vi "Dresden R2R Sputter 03.02.2018 IY24.vi"() -> ()   [LabVIEW 2009] (continued)
              frame #0 {
                n9135 = Wait (ms)(milliseconds to wait=i32? 100) -> ()  [unwired: 1 out]
              }
            }
            "Tp4_stop_cmnd" <- T/1 ("Tp4_stop_cmnd")
          }
          frame #3 {
            # "Address"
            n9136 = Multiply(x="Low_speed_value 4", y=data[16B]) -> (x*y=w14842)
            n9137 = To Unsigned Long Integer(number=w14842) -> (unsigned 32bit integer=w14841)
            n9138 = Number To Decimal String(number=w14841) -> (decimal integer string=w14839)  [unwired: 1 out]
            n9139 = String Length(string=w14839) -> (length=w14840)
            n9140 = case shown="0, Default" w14840 {
              tunnel: w14839 -> [_ w14868 w14871 w14872]
              tunnel: [data[5B] w14867 w14870 w14872] -> w14838
              frame #0 {
              }
              frame #1 {
                n9141 = Concatenate Strings(w14868, "00" ("string")) -> (w14867)
              }
              frame #2 {
                n9142 = Concatenate Strings(w14871, "0" ("string")) -> (w14870)
              }
              frame #3 {
              }
            }
            n9143 = Concatenate Strings("004" ("write buffer"), "10" ("string"), "707" ("string"), "06" ("string"), "00" ("string"), w14838) -> (w14852)
            n9144 = String To Byte Array(string=w14852) -> (unsigned byte array=w14857)
            n9145 = for {
              tunnel: w14857 -> [w14886] mode=indexing
              shift-right: [w14884] -> w14859
              shift-left: i16? 0 -> [w14885]
              n9146 = Add(x=w14886, y=w14885) -> (x+y=w14884)
            }
            n9147 = Number To Decimal String(number=w14859) -> (decimal integer string=w14854)  [unwired: 1 in]
            n9148 = String Length(string=w14854) -> (length=w14855)
            n9149 = case shown="0, Default" w14855 {
              tunnel: w14854 -> [_ w14879 w14882 w14883]
              tunnel: [data[5B] w14877 w14880 w14883] -> w14853
              frame #0 {
              }
              frame #1 {
                n9150 = Concatenate Strings("00" ("string"), w14879) -> (w14877)
              }
              frame #2 {
                n9151 = Concatenate Strings("0" ("string"), w14882) -> (w14880)
              }
              frame #3 {
              }
            }
            n9152 = Concatenate Strings(w14852, w14853, "\n") -> (w14849)
            n9153 = VISA Write(VISA resource name=w14848, write buffer=w14849, error in (no error)=w14847) -> (VISA resource name out=w14851, error out=w14850)  [unwired: 1 out]
            n9154 = stacked-sequence {
              tunnel: [w14875] -> w14846
              tunnel: w14851 -> [w14875]
              tunnel: [w14874] -> w14845
              tunnel: w14850 -> [w14874]
              frame #0 {
                n9155 = Wait (ms)(milliseconds to wait=i32? 100) -> ()  [unwired: 1 out]
              }
            }
          }
          frame #4 {
            # "Cheksum 3 haneli olmalı"
            # "Address"
            n9156 = Concatenate Strings("004" ("write buffer"), "10" ("string"), "026" ("string"), "03" ("string"), "001" ("string")) -> (w14894)
            n9157 = String To Byte Array(string=w14894) -> (unsigned byte array=w14899)
            n9158 = for {
              tunnel: w14899 -> [w14920] mode=indexing
              shift-right: [w14918] -> w14901
              shift-left: i16? 0 -> [w14919]
              n9159 = Add(x=w14920, y=w14919) -> (x+y=w14918)
            }
            n9160 = Number To Decimal String(number=w14901) -> (decimal integer string=w14896)  [unwired: 1 in]
            n9161 = String Length(string=w14896) -> (length=w14897)
            n9162 = case shown="0, Default" w14897 {
              tunnel: w14896 -> [_ w14913 w14916 w14917]
              tunnel: [data[5B] w14911 w14914 w14917] -> w14895
              frame #0 {
              }
              frame #1 {
                n9163 = Concatenate Strings("00" ("string"), w14913) -> (w14911)
              }
              frame #2 {
                n9164 = Concatenate Strings("0" ("string"), w14916) -> (w14914)
              }
              frame #3 {
              }
            }
            n9165 = Concatenate Strings(w14894, w14895, "\n") -> (w14891)
            n9166 = VISA Write(VISA resource name=w14890, write buffer=w14891, error in (no error)=w14889) -> (VISA resource name out=w14893, error out=w14892)  [unwired: 1 out]
            n9167 = stacked-sequence {
              tunnel: [w14909] -> w14888
              tunnel: w14893 -> [w14909]
              tunnel: [w14908] -> w14887
              tunnel: w14892 -> [w14908]
              frame #0 {
                n9168 = Wait (ms)(milliseconds to wait=i32? 100) -> ()  [unwired: 1 out]
              }
            }
          }
          frame #5 {
            # "Cheksum 3 haneli olmalı"
            # "Address"
            n9169 = Concatenate Strings("004" ("write buffer"), "10" ("string"), "026" ("string"), "03" ("string"), "000" ("string")) -> (w14928)
            n9170 = String To Byte Array(string=w14928) -> (unsigned byte array=w14933)
            n9171 = for {
              tunnel: w14933 -> [w14954] mode=indexing
              shift-right: [w14952] -> w14935
              shift-left: i16? 0 -> [w14953]
              n9172 = Add(x=w14954, y=w14953) -> (x+y=w14952)
            }
            n9173 = Number To Decimal String(number=w14935) -> (decimal integer string=w14930)  [unwired: 1 in]
            n9174 = String Length(string=w14930) -> (length=w14931)
            n9175 = case shown="0, Default" w14931 {
              tunnel: w14930 -> [_ w14947 w14950 w14951]
              tunnel: [data[5B] w14945 w14948 w14951] -> w14929
              frame #0 {
              }
              frame #1 {
                n9176 = Concatenate Strings("00" ("string"), w14947) -> (w14945)
              }
              frame #2 {
                n9177 = Concatenate Strings("0" ("string"), w14950) -> (w14948)
              }
              frame #3 {
              }
            }
            n9178 = Concatenate Strings(w14928, w14929, "\n") -> (w14925)
            n9179 = VISA Write(VISA resource name=w14924, write buffer=w14925, error in (no error)=w14923) -> (VISA resource name out=w14927, error out=w14926)  [unwired: 1 out]
            n9180 = stacked-sequence {
              tunnel: [w14943] -> w14922
              tunnel: w14927 -> [w14943]
              tunnel: [w14942] -> w14921
              tunnel: w14926 -> [w14942]
              frame #0 {
                n9181 = Wait (ms)(milliseconds to wait=i32? 100) -> ()  [unwired: 1 out]
              }
            }
          }
          frame #6 {
            # "Cheksum 3 haneli olmalı"
            # "Address"
            n9182 = Concatenate Strings("004" ("write buffer"), "10" ("string"), "023" ("string"), "06" ("string"), "111111" ("string")) -> (w14962)
            n9183 = String To Byte Array(string=w14962) -> (unsigned byte array=w14967)
            n9184 = for {
              tunnel: w14967 -> [w14988] mode=indexing
              shift-right: [w14986] -> w14969
              shift-left: i16? 0 -> [w14987]
              n9185 = Add(x=w14988, y=w14987) -> (x+y=w14986)
            }
            n9186 = Number To Decimal String(number=w14969) -> (decimal integer string=w14964)  [unwired: 1 in]
            n9187 = String Length(string=w14964) -> (length=w14965)
            n9188 = case shown="0, Default" w14965 {
              tunnel: w14964 -> [_ w14981 w14984 w14985]
              tunnel: [data[5B] w14979 w14982 w14985] -> w14963
              frame #0 {
              }
              frame #1 {
                n9189 = Concatenate Strings("00" ("string"), w14981) -> (w14979)
              }
              frame #2 {
                n9190 = Concatenate Strings("0" ("string"), w14984) -> (w14982)
              }
              frame #3 {
              }
            }
            n9191 = Concatenate Strings(w14962, w14963, "\n") -> (w14959)
            n9192 = VISA Write(VISA resource name=w14958, write buffer=w14959, error in (no error)=w14957) -> (VISA resource name out=w14961, error out=w14960)  [unwired: 1 out]
            n9193 = stacked-sequence {
              tunnel: [w14977] -> w14956
              tunnel: w14961 -> [w14977]
              tunnel: [w14976] -> w14955
              tunnel: w14960 -> [w14976]
              frame #0 {
                n9194 = Wait (ms)(milliseconds to wait=i32? 100) -> ()  [unwired: 1 out]
              }
            }
          }
          frame #7 {
            # "Cheksum 3 haneli olmalı"
            # "Address"
            n9195 = Concatenate Strings("004" ("write buffer"), "10" ("string"), "023" ("string"), "06" ("string"), "000000" ("string")) -> (w14996)
            n9196 = String To Byte Array(string=w14996) -> (unsigned byte array=w15001)
            n9197 = for {
              tunnel: w15001 -> [w15022] mode=indexing
              shift-right: [w15020] -> w15003
              shift-left: i16? 0 -> [w15021]
              n9198 = Add(x=w15022, y=w15021) -> (x+y=w15020)
            }
            n9199 = Number To Decimal String(number=w15003) -> (decimal integer string=w14998)  [unwired: 1 in]
            n9200 = String Length(string=w14998) -> (length=w14999)
            n9201 = case shown="0, Default" w14999 {
              tunnel: w14998 -> [_ w15015 w15018 w15019]
              tunnel: [data[5B] w15013 w15016 w15019] -> w14997
              frame #0 {
              }
              frame #1 {
                n9202 = Concatenate Strings("00" ("string"), w15015) -> (w15013)
              }
              frame #2 {
                n9203 = Concatenate Strings("0" ("string"), w15018) -> (w15016)
              }
              frame #3 {
              }
            }
            n9204 = Concatenate Strings(w14996, w14997, "\n") -> (w14993)
            n9205 = VISA Write(VISA resource name=w14992, write buffer=w14993, error in (no error)=w14991) -> (VISA resource name out=w14995, error out=w14994)  [unwired: 1 out]
            n9206 = stacked-sequence {
              tunnel: [w15011] -> w14990
              tunnel: w14995 -> [w15011]
              tunnel: [w15010] -> w14989
              tunnel: w14994 -> [w15010]
              frame #0 {
                n9207 = Wait (ms)(milliseconds to wait=i32? 100) -> ()  [unwired: 1 out]
              }
            }
          }
        }
      }
    }
  }
  n9208 = while {
    tunnel: w749 -> [w15026]
    tunnel: w775 -> [w15025]
    tunnel: [w15029] -> w774
    tunnel: [w15024] -> w743
    tunnel: "milliseconds to wait 2" -> [w15023]
    stop <- FALSE stop-if-true
    n9209 = stacked-sequence {
      tunnel: w15025 -> [w15034 _]
      tunnel: [w15033 _] -> w15029
      tunnel: w15026 -> [w15032 _]
      tunnel: [w15031 _] -> w15024
      tunnel: w15023 -> [w15030 _]
      frame #0 {
        n9210 = stacked-sequence {
          tunnel: w15032 -> [w15045 _ _ _ _ _ _ _ _]
          tunnel: w15034 -> [w15044 _ _ _ _ _ _ _ _]
          tunnel: [_ _ _ w15171 _ _ _ _ _] -> w15031
          tunnel: [_ _ _ w15169 _ _ _ _ _] -> w15033
          tunnel: w15030 -> [_ _ w15168 _ w15249 _ w15409 _ w15446]
          frame #0 {
            # "Digital I/O & Analog \nOutput Part"
            n9211 = disable-structure shown="Enabled" {
              disable-tunnel: w15045 -> [w15146 w15148]
              disable-tunnel: w15044 -> [w15145 w15147]
              disable-tunnel: [w15127 w15148] -> w15043
              disable-tunnel: [w15126 w15147] -> w15042
              frame #0 {
                n9212 = call-poly <vilib>:"MB Serial Master Query (poly).vi"("VISA resource name"=w15146, "Starting Address"=u16 0, "Quantity"=u16 8, "error in"=w15145, "Serial Parameters"=T39 {"Mode"=enum."RTU", "Slave Address"=1}) -> ("VISA resource name out"=w15127:refnum<visa-resource-name>, "Discrete Inputs"=w15135:bool[], "error out"=w15126:errorcluster)  [unwired: 1 in, 11 out]
                n9213 = Index Array(array=w15135, index=5) -> (element=w15125:bool)
                "Ch1_Pl_vbv_di" <- w15125
                n9214 = Index Array(array=w15135, index=6) -> (element=w15130:bool)
                "Ch1_Pl_atm_di" <- w15130
                n9215 = Index Array(array=w15135, index=7) -> (element=w15123:bool)
                "Ch1_Cc_on_off_di" <- w15123
                n9216 = Index Array(array=w15135, index=0) -> (element=w15133:bool)
                "Ch1_Mp_di" <- w15133
                n9217 = Index Array(array=w15135, index=1) -> (element=w15129:bool)
                "Ch1_Tp_bv_di" <- w15129
                n9218 = Index Array(array=w15135, index=2) -> (element=w15124:bool)
                "Ch1_Bg_bv_di" <- w15124
                n9219 = Index Array(array=w15135, index=3) -> (element=w15132:bool)
                "Ch1_Ch_vbv_di" <- w15132
                n9220 = Index Array(array=w15135, index=4) -> (element=w15131:bool)
                "Ch1_Ch_atm_di" <- w15131
                n9221 = local write "ch1_bg_bv_on_top"(w15124) -> ()
                n9222 = local write "Ch1_Ch_vbv_on"(w15132) -> ()
                n9223 = local write "ch4_atm_on_top"(w15131) -> ()
                n9224 = local write "Ch1_Ch_atm_on"(w15131) -> ()
                n9225 = local write "Ch1_Mp_on"(w15133) -> ()
                n9226 = local write "Ch1_Tp_bv_on"(w15129) -> ()
                n9227 = local write "Ch1_Bg_bv_on"(w15124) -> ()
                n9228 = local write "Ch1_Pl_vbv_on"(w15125) -> ()
                n9229 = local write "Ch1_Pl_atm_on"(w15130) -> ()
                n9230 = local write "Ch1_Ch_cc_on"(w15123) -> ()
                n9231 = local write "ch1_cc_on_top"(w15123) -> ()
              }
              frame #1 {
              }
            }
            n9232 = disable-structure shown="Enabled" {
              disable-tunnel: w15043 -> [w15104 w15122]
              disable-tunnel: w15042 -> [w15102 w15121]
              disable-tunnel: [w15101 w15122] -> w15041
              disable-tunnel: [w15100 w15121] -> w15040
              frame #0 {
                n9233 = call-poly <vilib>:"MB Serial Master Query (poly).vi"("VISA resource name"=w15104, "Starting Address"=u16 0, "Quantity"=u16 8, "error in"=w15102, "Serial Parameters"=T39 {"Mode"=enum."RTU", "Slave Address"=2}) -> ("VISA resource name out"=w15101:refnum<visa-resource-name>, "Discrete Inputs"=w15114:bool[], "error out"=w15100:errorcluster)  [unwired: 1 in, 11 out]
                n9234 = Index Array(array=w15114, index=5) -> (element=w15098:bool)
                "Ch1_Cst_fix_down_di" <- w15098
                n9235 = Index Array(array=w15114, index=6) -> (element=→"Ch1_Pet_cool_up_di":bool)
                n9236 = Index Array(array=w15114, index=7) -> (element=→"Ch1_Pet_cool_down_di":bool)
                n9237 = Index Array(array=w15114, index=0) -> (element=w15099:bool)
                "Ch1_Sov_Ar_di" <- w15099
                n9238 = Index Array(array=w15114, index=1) -> (element=w15097:bool)
                "Ch1_Trns_gv_open_di" <- w15097
                n9239 = Index Array(array=w15114, index=2) -> (element=→"Ch1_Trns_gv_close_di":bool)
                n9240 = Index Array(array=w15114, index=3) -> (element=→"Ch1_2_3_di":bool)
                n9241 = Index Array(array=w15114, index=4) -> (element=→"Ch1_Cst_fix_up_di":bool)
                n9242 = local write "chamber 1 top piston open ch1"(w15098) -> ()
                n9243 = local write "ch1_sov_Ar_on_top"(w15099) -> ()
                n9244 = local write "gv front open ch1_2"(w15097) -> ()
                n9245 = local write "Trns_gv_1_2_on"(w15097) -> ()
                n9246 = local write "gv top open ch1"(w15097) -> ()
                n9247 = local write "gv front open_ch2_1"(w15097) -> ()
                n9248 = local write "gv top_open_ch2_1"(w15097) -> ()
              }
              frame #1 {
              }
            }
            n9249 = local read "Load_dido"() -> (w15035:bool)
            n9250 = case shown="True" w15035 {
              frame #0 {
              }
              frame #1 {
                n9251 = Wait (ms)(milliseconds to wait=u32 2000) -> ()  [unwired: 1 out]
              }
            }
            n9252 = disable-structure shown="Enabled" {
              disable-tunnel: w15041 -> [w15052 w15070]
              disable-tunnel: w15040 -> [w15051 w15069]
              disable-tunnel: [w15050 w15070] -> w15039
              disable-tunnel: [w15049 w15069] -> w15038
              frame #0 {
                n9253 = call-poly <vilib>:"MB Serial Master Query (poly).vi"("VISA resource name"=w15052, "Starting Address"=u16 0, "Quantity"=u16 8, "error in"=w15051, "Serial Parameters"=T39 {"Mode"=enum."RTU", "Slave Address"=3}) -> ("VISA resource name out"=w15050:refnum<visa-resource-name>, "Discrete Inputs"=w15046:bool[], "error out"=w15049:errorcluster)  [unwired: 1 in, 11 out]
                n9254 = Index Array(array=w15046, index=3) -> ()  [unwired: 1 out]
                n9255 = Index Array(array=w15046, index=5) -> (element=→"Ch1_SRV2_counter_di":bool)
                n9256 = Index Array(array=w15046, index=6) -> (element=→"Ch1_WFS_di":bool)
                n9257 = Index Array(array=w15046, index=7) -> (element=w15048:bool)
                "Ch1_Trns_gv_bp2_di" <- w15048
                n9258 = Index Array(array=w15046, index=0) -> (element=→"Ch1_SRV1_PIST For_di":bool)
                n9259 = Index Array(array=w15046, index=1) -> (element=→"Ch1_SRV1_PIST_Back_di":bool)
                n9260 = Index Array(array=w15046, index=2) -> (element=→"Ch1_SRV_start_stop_di":bool)
                n9261 = Index Array(array=w15046, index=3) -> (element=→"Ch1_SRV_left_direction_di":bool)
                n9262 = local write "Ch1_Trns_gv_bp2_on"(w15048) -> ()
                n9263 = local write "Trns_gv_bp2_ch1_on_top"(w15048) -> ()
                n9264 = local write "Trns_gv_bp2_ch1_on_front"(w15048) -> ()
              }
              frame #1 {
              }
            }
            n9265 = disable-structure shown="Enabled" {
              disable-tunnel: w15039 -> [w15075 w15096]
              disable-tunnel: w15038 -> [w15074 w15095]
              disable-tunnel: [w15073 w15096] -> w15037
              disable-tunnel: [w15072 w15095] -> w15036
              frame #0 {
                n9266 = call-poly <vilib>:"MB Serial Master Query (poly).vi"("VISA resource name"=w15075, "Starting Address"=u16 0, "Quantity"=u16 8, "error in"=w15074, "Serial Parameters"=T39 {"Mode"=enum."RTU", "Slave Address"=4}) -> ("VISA resource name out"=w15073:refnum<visa-resource-name>, "Discrete Inputs"=w15092:bool[], "error out"=w15072:errorcluster)  [unwired: 1 in, 11 out]
                n9267 = Index Array(array=w15092, index=5) -> (element=→"Ch1_Right_slow_di":bool)
                n9268 = Index Array(array=w15092, index=6) -> (element=→"Ch1_4_6_di":bool)
                n9269 = Index Array(array=w15092, index=7) -> (element=→"Ch1_4_7_di":bool)
                n9270 = Index Array(array=w15092, index=0) -> (element=→"Ch1_Air_press_di":bool)
                n9271 = Index Array(array=w15092, index=1) -> (element=→"Ch1_Ds_di":bool)
                n9272 = Index Array(array=w15092, index=2) -> (element=→"Ch1_TGV_control_di":bool)
                n9273 = Index Array(array=w15092, index=3) -> (element=→"Ch1_Trns_interlock_di":bool)
                n9274 = Index Array(array=w15092, index=4) -> (element=→"Ch1_Right_limit_di":bool)
              }
              frame #1 {
              }
            }
          }
          frame #1 {
            n9275 = local read "Load_dido"() -> (w15150:bool)
            n9276 = case shown="True" w15150 {
              frame #0 {
              }
              frame #1 {
                n9277 = while {
                  stop <- w15161 stop-if-true
                  n9278 = local read "Ch1_Pl_vbv_di"() -> (w15163:bool)
                  n9279 = local read "Ch1_Mp_di"() -> (w15167:bool)
                  n9280 = local read "Ch1_Tp_bv_di"() -> (w15166:bool)
                  n9281 = local read "Ch1_Bg_bv_di"() -> (w15165:bool)
                  n9282 = local read "Ch1_Ch_vbv_di"() -> (w15164:bool)
                  n9283 = local read "Ch1_Cc_on_off_di"() -> (w15162:bool)
                  n9284 = Wait Until Next ms Multiple(millisecond multiple=u32 300) -> ()  [unwired: 1 out]
                  n9285 = local write "Ch1_Mp_do"(w15167) -> ()
                  n9286 = local write "Ch1_Tp_bv_do"(w15166) -> ()
                  n9287 = local write "Ch1_Bg_bv_do"(w15165) -> ()
                  n9288 = local write "Ch1_Ch_vbv_do"(w15164) -> ()
                  n9289 = local write "Ch1_Pl_vbv_do"(w15163) -> ()
                  n9290 = local write "Ch1_Cc_on_off_do"(w15162) -> ()
                  n9291 = local read "Ch1_Cst_fix_down_di"() -> (w15156:bool)
                  n9292 = local read "Ch1_Sov_Ar_di"() -> (w15153:bool)
                  n9293 = local read "Ch1_Trns_gv_open_di"() -> (w15154:bool)
                  n9294 = local read "Ch1_Trns_gv_close_di"() -> (w15155:bool)
                  n9295 = local read "Ch1_Pet_cool_up_di"() -> (w15157:bool)
                  n9296 = local read "Ch1_Pet_cool_down_di"() -> (w15158:bool)
                  n9297 = local write "Ch1_Sov_Ar_do"(w15153) -> ()
                  n9298 = local write "Ch1_Trns_gv_open_do"(w15154) -> ()
                  n9299 = local write "Ch1_Trns_gv_close_do"(w15155) -> ()
                  n9300 = local write "Ch1_Pet_cool_up_do"(w15157) -> ()
                  n9301 = local write "Ch1_Pet_cool_down_do"(w15158) -> ()
                  n9302 = local write "Ch1_Cst_fix_do"(w15156) -> ()
                  n9303 = local read "Ch1_Trns_gv_bp2_di"() -> (w15151:bool)
                  n9304 = local read "Load_dido"() -> (w15160:bool)
                  n9305 = local read "Ch1_WFS_di"() -> (w15152:bool)
                  n9306 = local write "Ch1_Trns_gv_bp2_do"(w15151) -> ()
                  n9307 = Not(x=w15160) -> (.not. x?=w15161:bool)
                  n9308 = local write "Ch1_WFC_do"(w15152) -> ()
                }
              }
            }
          }
          frame #2 {
            n9309 = Wait (ms)(milliseconds to wait=w15168) -> ()  [unwired: 1 out]
          }
          frame #3 {
            n9310 = disable-structure shown="Enabled" {
              disable-tunnel: w15176 -> [w15235 w15247]
              disable-tunnel: [w15234 w15247] -> w15175
              disable-tunnel: w15173 -> [_ w15248]
              disable-tunnel: [w15233 w15248] -> w15174
              frame #0 {
                n9311 = Build Array("Ch1_Mp_do", "Ch1_Tp_bv_do", "Ch1_Bg_bv_do", "Ch1_Ch_vbv_do", "Ch1_Ch_atm_do", "Ch1_Pl_vbv_do", "Ch1_Pl_atm_do", "Ch1_Cc_on_off_do") -> (w15237:bool[])
                n9312 = call-poly <vilib>:"MB Serial Master Query (poly).vi"("VISA resource name"=w15235, "Starting Address"=u16 320, "Coils"=w15237, "Serial Parameters"=T39 {"Mode"=enum."RTU", "Slave Address"=1}) -> ("VISA resource name out"=w15234:refnum<visa-resource-name>, "error out"=w15233:errorcluster)  [unwired: 2 in, 12 out]
              }
              frame #1 {
              }
            }
            n9313 = call "Elapsed Time146"() -> ("Elapsed Time (s)"=w15179:dbl)  [unwired: 12 in, 7 out]
            "COM12 Time" <- w15179
            n9314 = feedback #281() -> (w15180:dbl)  [unwired: 1 in]
            n9315 = Subtract(x=w15179, y=w15180) -> (x-y=→"COM12 Loop Time":dbl)
            n9316 = disable-structure shown="Enabled" {
              disable-tunnel: [w15201 w15215] -> w15178
              disable-tunnel: w15175 -> [w15202 w15215]
              disable-tunnel: [w15200 w15214] -> w15177
              disable-tunnel: w15174 -> [w15199 w15214]
              frame #0 {
                n9317 = Build Array("Ch1_Sov_Ar_do", "Ch1_Trns_gv_open_do", "Ch1_Trns_gv_close_do", "Ch1_2_3_do", "Ch1_Cst_fix_do", "Ch1_2_5_di", "Ch1_Pet_cool_up_do", "Ch1_Pet_cool_down_do") -> (w15204:bool[])
                n9318 = call-poly <vilib>:"MB Serial Master Query (poly).vi"("VISA resource name"=w15202, "Starting Address"=u16 320, "Coils"=w15204, "error in"=w15199, "Serial Parameters"=T39 {"Mode"=enum."RTU", "Slave Address"=2}) -> ("VISA resource name out"=w15201:refnum<visa-resource-name>, "error out"=w15200:errorcluster)  [unwired: 1 in, 12 out]
              }
              frame #1 {
              }
            }
            n9319 = disable-structure shown="Enabled" {
              disable-tunnel: w15178 -> [w15186 w15198]
              disable-tunnel: w15177 -> [w15185 w15197]
              disable-tunnel: [w15184 w15198] -> w15172
              disable-tunnel: [w15183 w15197] -> w15170
              frame #0 {
                n9320 = Build Array("Ch1_SRV1_PIST For_do", "Ch1_SRV1_PIST_Back_do", "Ch1_3_2_do", "Ch1_SRV_counterclockwise_direction_do", "Ch1_3_4_do", "Ch1_3_5_do", "Ch1_WFC_do", "Ch1_Trns_gv_bp2_do") -> (w15189:bool[])
                n9321 = call-poly <vilib>:"MB Serial Master Query (poly).vi"("VISA resource name"=w15186, "Starting Address"=u16 320, "Coils"=w15189, "error in"=w15185, "Serial Parameters"=T39 {"Mode"=enum."RTU", "Slave Address"=3}) -> ("VISA resource name out"=w15184:refnum<visa-resource-name>, "error out"=w15183:errorcluster)  [unwired: 1 in, 12 out]
              }
              frame #1 {
              }
            }
            n9322 = disable-structure shown="Enabled" {
              disable-tunnel: w15172 -> [w15219 w15232]
              disable-tunnel: [w15218 w15232] -> w15171
              disable-tunnel: w15170 -> [w15217 w15231]
              disable-tunnel: [w15216 w15231] -> w15169
              frame #0 {
                n9323 = Build Array("Ch1_Do_4_0", "Ch1_Do_4_1", "Ch1_TGV_control_do", "Ch1_Do_4_3", "Ch1_Do_4_4", "Ch1_Do_4_5", "Ch1_Do_4_6", "Ch1_Do_4_7") -> (w15221:bool[])
                n9324 = call-poly <vilib>:"MB Serial Master Query (poly).vi"("VISA resource name"=w15219, "Starting Address"=u16 320, "Coils"=w15221, "error in"=w15217, "Serial Parameters"=T39 {"Mode"=enum."RTU", "Slave Address"=4}) -> ("VISA resource name out"=w15218:refnum<visa-resource-name>, "error out"=w15216:errorcluster)  [unwired: 1 in, 12 out]
              }
              frame #1 {
              }
            }
          }
          frame #4 {
            n9325 = Wait (ms)(milliseconds to wait=w15249) -> ()  [unwired: 1 out]
          }
          frame #5 {
            n9326 = disable-structure shown="Disabled" {
              disable-tunnel: [w15254 _] -> _
              disable-tunnel: [w15253 _] -> _
              frame #0 {
                n9327 = call-poly <vilib>:"MB Serial Master Query (poly).vi"("Starting Address"=u16 704, "Quantity"=u16 8, "Serial Parameters"=T39 {"Mode"=enum."RTU", "Slave Address"=5}) -> ("VISA resource name out"=w15254:refnum<visa-resource-name>, "Input Registers"=w15268:u16[], "error out"=w15253:errorcluster)  [unwired: 3 in, 11 out]
                n9328 = local read "1bit="() -> (w15256:dbl)
                n9329 = local read "1bit="() -> (w15258:dbl)
                n9330 = Index Array(array=w15268, index=5) -> (element=→"Ch1_Ai_1_5":u16)
                n9331 = Index Array(array=w15268, index=6) -> (element=→"Ch1_Ai_1_6":u16)
                n9332 = Index Array(array=w15268, index=7) -> (element=→"Ch1_Ai_1_7":u16)
                n9333 = Index Array(array=w15268, index=0) -> (element=w15260:u16)
                "Ch1_Ai_PL_PG" <- w15260
                n9334 = Index Array(array=w15268, index=1) -> (element=w15251:u16)
                "Ch1_Ai_CH_PG" <- w15251
                n9335 = Multiply(x=w15258, y=w15251) -> (x*y=w15257:dbl)
                n9336 = stacked-sequence {
                  tunnel: w15257 -> [w15346]
                  frame #0 {
                    # "CH-PG 0-10 Volt okuma"
                    n9337 = feedback #282() -> (w15357:dbl)  [unwired: 1 in]
                    n9338 = feedback #283() -> (w15355:dbl)  [unwired: 1 in]
                    n9339 = feedback #284() -> (w15354:dbl)  [unwired: 1 in]
                    n9340 = feedback #285() -> (w15353:dbl)  [unwired: 1 in]
                    n9341 = feedback #286() -> (w15352:dbl)  [unwired: 1 in]
                    n9342 = feedback #287() -> (w15351:dbl)  [unwired: 1 in]
                    n9343 = feedback #288() -> (w15350:dbl)  [unwired: 1 in]
                    n9344 = feedback #289() -> (w15348:dbl)  [unwired: 1 in]
                    n9345 = feedback #290() -> (w15349:dbl)  [unwired: 1 in]
                    n9346 = Compound Arithmetic op=ADD(w15346, w15357, w15355, w15354, w15353, w15352, w15351, w15350, w15348, w15349) -> (w15356:dbl)
                    n9347 = local read "Ch_pg_volt_instantaneous_ch1"() -> (w15339:dbl)
                    n9348 = Divide(x=w15356, y=u16 10) -> (x/y=w15340:dbl)
                    "Ch_pg_volt_ch1" <- w15340
                    n9349 = Greater Or Equal?(x=w15339, y=u16 1) -> (x >= y?=w15341:bool)
                    n9350 = feedback #291() -> (w15344:bool)  [unwired: 1 in]
                    n9351 = case shown="True" w15341 {
                      tunnel: w15340 -> [_ w15369]
                      tunnel: [FALSE TRUE] -> w15343
                      tunnel: w15344 -> [w15360 _]
                      tunnel: [w15359 FALSE ("Bg_gui")] -> w15345
                      frame #0 {
                        n9352 = local write "Ch3_Ch_pg_on"(FALSE ("Bg_gui")) -> ()
                        n9353 = call "Elapsed Time142"("Reset"=w15360) -> ("Elapsed Time (s)"=w15363:dbl)  [unwired: 11 in, 7 out]
                        n9354 = Greater Or Equal?(x=w15363, y=3.0) -> (x >= y?=w15359:bool)
                      }
                      frame #1 {
                        n9355 = Subtract(x=w15369, y=5.625) -> (x-y=w15371:dbl)
                        n9356 = Power Of 10(x=w15371) -> (10^x=w15370:dbl)
                        n9357 = In Range and Coerce(upper limit=760.0, x=w15370, lower limit=0.000375) -> (coerced(x)=→"Ch_pg_press_ch1" →"Ch_pg_press_ch1_gui" →"Ch_pg_press_ch1_gui 2":dbl)  [unwired: 1 out]
                        n9358 = local write "Ch1_Ch_pg_on"(TRUE ("Bg_gui")) -> ()
                      }
                    }
                    n9359 = local write "Ch1_Ch_pg_fail"(w15345) -> ()
                    "Ch_pg_volt_instantaneous_ch1" <- w15346
                  }
                }
                n9360 = Index Array(array=w15268, index=2) -> (element=w15252:u16)
                "Ch1_Ai_CH-CC" <- w15252
                n9361 = Multiply(x=w15256, y=w15252) -> (x*y=w15255:dbl)
                n9362 = stacked-sequence {
                  tunnel: w15255 -> [w15310]
                  frame #0 {
                    # "CH-CC 0-10 Volt okuma"
                    n9363 = feedback #292() -> (w15311:dbl)  [unwired: 1 in]
                    n9364 = feedback #293() -> (w15312:dbl)  [unwired: 1 in]
                    n9365 = feedback #294() -> (w15313:dbl)  [unwired: 1 in]
                    n9366 = feedback #295() -> (w15314:dbl)  [unwired: 1 in]
                    n9367 = feedback #296() -> (w15315:dbl)  [unwired: 1 in]
                    n9368 = feedback #297() -> (w15316:dbl)  [unwired: 1 in]
                    n9369 = feedback #298() -> (w15317:dbl)  [unwired: 1 in]
                    n9370 = feedback #299() -> (w15318:dbl)  [unwired: 1 in]
                    n9371 = feedback #300() -> (w15301:dbl)  [unwired: 1 in]
                    n9372 = feedback #301() -> (w15300:dbl)  [unwired: 1 in]
                    n9373 = feedback #302() -> (w15299:dbl)  [unwired: 1 in]
                    n9374 = feedback #303() -> (w15298:dbl)  [unwired: 1 in]
                    n9375 = feedback #304() -> (w15297:dbl)  [unwired: 1 in]
                    n9376 = feedback #305() -> (w15296:dbl)  [unwired: 1 in]
                    n9377 = feedback #306() -> (w15295:dbl)  [unwired: 1 in]
                    n9378 = feedback #307() -> (w15294:dbl)  [unwired: 1 in]
                    n9379 = feedback #308() -> (w15293:dbl)  [unwired: 1 in]
                    n9380 = feedback #309() -> (w15292:dbl)  [unwired: 1 in]
                    n9381 = feedback #310() -> (w15291:dbl)  [unwired: 1 in]
                    n9382 = Compound Arithmetic op=ADD(w15310, w15311, w15312, w15313, w15314, w15315, w15316, w15317, w15318, w15301, w15300, w15299, w15298, w15297, w15296, w15295, w15294, w15293, w15292, w15291) -> (w15309:dbl)
                    n9383 = Divide(x=w15309, y=u16 20) -> (x/y=w15305:dbl)
                    "Ch_CC_volt_ch1" <- w15305
                    n9384 = Greater?(x=w15305, y=1.0) -> (0:w15306:bool)
                    n9385 = feedback #311() -> (w15302:bool)  [unwired: 1 in]
                    n9386 = case shown="True" w15306 {
                      tunnel: w15305 -> [_ w15335]
                      tunnel: [w15326 FALSE] -> w15304
                      tunnel: [FALSE ("Ch_cc_on(ch1)") TRUE] -> w15303
                      tunnel: w15302 -> [_ _]
                      frame #0 {
                        n9387 = local read "Ch1_Cc_on_off_di"() -> (w15320:bool)
                        n9388 = call "Elapsed Time84"() -> ("Elapsed Time (s)"=w15329:dbl)  [unwired: 12 in, 7 out]
                        n9389 = Not(x=w15320) -> (.not. x?=w15323:bool)
                        n9390 = Greater Or Equal?(x=w15329, y=3.0) -> (x >= y?=w15328:bool)
                        n9391 = call "Elapsed Time85"("Reset"=w15323) -> ("Elapsed Time (s)"=w15325:dbl)  [unwired: 11 in, 7 out]
                        n9392 = local write "Ch1_Ch_cc_on"(FALSE ("Ch_cc_on(ch1)")) -> ()
                        n9393 = Greater Or Equal?(x=w15325, y=3.0) -> (x >= y?=w15322:bool)
                        n9394 = And(x=w15328, y=w15322) -> (x .and. y?=w15326:bool)
                      }
                      frame #1 {
                        n9395 = Subtract(x=w15335, y=10.625) -> (x-y=w15332:dbl)
                        n9396 = Power Of 10(x=w15332) -> (10^x=w15331:dbl)
                        n9397 = In Range and Coerce(upper limit=0.0075, x=w15331, lower limit=1.5e-09) -> (coerced(x)=→"Ch_CC_press_ch1_gui1" →"Ch_CC_press_ch1" →"Ch_CC_press_ch1_gui1 2":dbl)  [unwired: 1 out]
                      }
                    }
                    n9398 = local write "Ch1_Ch_cc_fail"(w15304) -> ()
                  }
                }
                n9399 = Index Array(array=w15268, index=3) -> (element=→"Ch1_Ai_1_3":u16)
                n9400 = Index Array(array=w15268, index=4) -> (element=→"Ch1_Ai_1_4":u16)
                n9401 = Divide(x=10.0, y=65536.0) -> (x/y=w15261:dbl)
                "1bit=" <- w15261
                n9402 = Multiply(x=w15261, y=w15260) -> (x*y=w15259:dbl)
                n9403 = stacked-sequence {
                  frame #0 {
                    n9404 = local read "Ch1_Cc_on_off_di"() -> (w15280:bool)
                    n9405 = case shown="False" w15280 {
                      frame #0 {
                        n9406 = local read "Ch_pg_press_ch1"() -> (→"Ch1_pressure 2" →"Ch1_pressure":dbl)
                      }
                      frame #1 {
                        n9407 = local read "Ch_CC_volt_ch1"() -> (w15288:dbl)
                        n9408 = local read "Ch_pg_volt_ch1"() -> (w15287:u16)
                        n9409 = Greater?(x=w15288, y=1.8) -> (0:w15286:bool)
                        n9410 = Less?(x=w15287, y=u16 2) -> (x < y?=w15285:bool)
                        n9411 = Or(x=w15286, y=w15285) -> (x .or. y?=w15284:bool)
                        n9412 = case shown="True" w15284 {
                          frame #0 {
                            n9413 = local read "Ch_pg_press_ch1"() -> (w15289:dbl)
                            n9414 = local write "Ch1_pressure"(w15289) -> ()
                            n9415 = local write "Ch1_pressure 2"(w15289) -> ()
                          }
                          frame #1 {
                            n9416 = local read "Ch_CC_press_ch1_gui1"() -> (w15290:dbl)
                            n9417 = local write "Ch1_pressure"(w15290) -> ()
                            n9418 = local write "Ch1_pressure 2"(w15290) -> ()
                          }
                        }
                      }
                    }
                  }
                }
                n9419 = stacked-sequence {
                  tunnel: w15259 -> [w15374]
                  frame #0 {
                    # "PL-PG 0-10 Volt okuma"
                    n9420 = feedback #312() -> (w15392:dbl)  [unwired: 1 in]
                    n9421 = feedback #313() -> (w15390:dbl)  [unwired: 1 in]
                    n9422 = feedback #314() -> (w15389:dbl)  [unwired: 1 in]
                    n9423 = feedback #315() -> (w15388:dbl)  [unwired: 1 in]
                    n9424 = feedback #316() -> (w15387:dbl)  [unwired: 1 in]
                    n9425 = feedback #317() -> (w15386:dbl)  [unwired: 1 in]
                    n9426 = feedback #318() -> (w15385:dbl)  [unwired: 1 in]
                    n9427 = feedback #319() -> (w15383:dbl)  [unwired: 1 in]
                    n9428 = feedback #320() -> (w15384:dbl)  [unwired: 1 in]
                    n9429 = Compound Arithmetic op=ADD(w15374, w15392, w15390, w15389, w15388, w15387, w15386, w15385, w15383, w15384) -> (w15391:dbl)
                    n9430 = local read "Pl_pg_volt_instantaneous_ch1"() -> (w15380:dbl)
                    n9431 = Divide(x=w15391, y=10.0) -> (x/y=w15381:dbl)
                    "Pl_pg_volt_ch1" <- w15381
                    n9432 = Greater Or Equal?(x=w15380, y=u16 1) -> (x >= y?=w15379:bool)
                    n9433 = feedback #321() -> (w15376:bool)  [unwired: 1 in]
                    n9434 = case shown="True" w15379 {
                      tunnel: w15381 -> [_ w15400]
                      tunnel: [FALSE TRUE] -> w15377
                      tunnel: w15376 -> [w15395 _]
                      tunnel: [w15394 FALSE ("Bg_gui")] -> w15375
                      frame #0 {
                        n9435 = local write "Ch1_Pl_pg_on"(FALSE ("Bg_gui")) -> ()
                        n9436 = call "Elapsed Time55"("Reset"=w15395) -> ("Elapsed Time (s)"=w15398:dbl)  [unwired: 11 in, 7 out]
                        n9437 = Greater Or Equal?(x=w15398, y=3.0) -> (x >= y?=w15394:bool)
                      }
                      frame #1 {
                        n9438 = Subtract(x=w15400, y=5.625) -> (x-y=w15399:dbl)
                        n9439 = Power Of 10(x=w15399) -> (10^x=w15406:dbl)
                        n9440 = local write "Ch1_Pl_pg_on"(TRUE ("Bg_gui")) -> ()
                        n9441 = In Range and Coerce(upper limit=760.0, x=w15406, lower limit=0.000375) -> (coerced(x)=→"Pl_pg_press_ch1" →"Pl_pg_press_ch1_gui":dbl)  [unwired: 1 out]
                      }
                    }
                    n9442 = local write "Ch1_Pl_pg_fail"(w15375) -> ()
                    "Pl_pg_volt_instantaneous_ch1" <- w15374
                  }
                }
              }
              frame #1 {
              }
            }
          }
          frame #6 {
            n9443 = Wait (ms)(milliseconds to wait=w15409) -> ()  [unwired: 1 out]
          }
          frame #7 {
            n9444 = disable-structure shown="Disabled" {
              disable-tunnel: [w15421 _] -> _
              disable-tunnel: [w15420 _] -> _
              frame #0 {
                n9445 = Build Array(FALSE, "Ch1_MW1_set", "Ch1_MW2_set", "Ch1_Ao_1_2", "Ch1_Ao_1_3") -> (w15416:bool[])
                n9446 = Boolean Array To Number(Boolean array=w15416) -> (number=w15419:u32)
                n9447 = Mantissa & Exponent(0:w15419) -> (2:w15415:dbl)  [unwired: 1 out]
                n9448 = case shown="1" w15415 {
                  tunnel: [u16 0 ("Starting Address") u16 1184 ("Starting Address") u16 1185 ("Starting Address") u16 1186 ("Starting Address") u16 1187 ("Starting Address")] -> w15422
                  tunnel: [u16 0 ("Ao_1_3") w15426 w15434 "Ch1_Ao_1_2" "Ch1_Ao_1_3 2"] -> w15414
                  frame #0 {
                  }
                  frame #1 {
                    n9449 = flat-sequence {
                      frame #0 {
                        n9450 = Wait (ms)(milliseconds to wait=u32 100) -> ()  [unwired: 1 out]
                      }
                      frame #1 {
                        n9451 = local write "Ch1_MW1_set"(FALSE ("Mfc_Ar _set")) -> ()
                      }
                    }
                    n9452 = Divide(x=2048, y=1500) -> (x/y=w15428:dbl)
                    n9453 = Multiply(x=w15428, y="Ch1_MW1") -> (x*y=w15426:dbl)
                  }
                  frame #2 {
                    n9454 = flat-sequence {
                      frame #0 {
                        n9455 = Wait (ms)(milliseconds to wait=u32 100) -> ()  [unwired: 1 out]
                      }
                      frame #1 {
                        n9456 = local write "Ch1_MW2_set"(FALSE ("Mfc_Ar _set")) -> ()
                      }
                    }
                    n9457 = Divide(x=2048.0, y=1500.0) -> (x/y=w15435:dbl)
                    n9458 = Multiply(x=w15435, y="Ch1_MW2") -> (x*y=w15434:dbl)
                  }
                  frame #3 {
                  }
                  frame #4 {
                  }
                }
                n9459 = Build Array(w15414) -> (w15413:dbl[])
                n9460 = call-poly <vilib>:"MB Serial Master Query (poly).vi"("Starting Address"=w15422, "Registers"=w15413, "Serial Parameters"=T39 {"Mode"=enum."RTU", "Slave Address"=6}) -> ("VISA resource name out"=w15421:refnum<visa-resource-name>, "error out"=w15420:errorcluster)  [unwired: 3 in, 12 out]
              }
              frame #1 {
              }
            }
          }
          frame #8 {
            n9461 = Wait (ms)(milliseconds to wait=w15446) -> ()  [unwired: 1 out]
          }
        }
      }
      frame #1 {
        n9462 = local read "Fail_moxa1_digital2"() -> (w15450:bool)
        n9463 = local read "Fail_moxa1_digital3"() -> (w15449:bool)
        n9464 = local read "Fail_moxa1_digital4"() -> (w15448:bool)
        n9465 = local read "Fail_moxa1_digital1"() -> (w15447:bool)
        n9466 = case shown="False" w15449 {
          frame #0 {
            n9467 = local read "Ch1_Trns_gv_bp2_do"() -> (w15466:bool)
            n9468 = local read "Ch1_Trns_gv_bp2_di"() -> (w15467:bool)
            n9469 = Exclusive Or(1:w15467, 2:w15466) -> (0:w15470:bool)
            n9470 = feedback #322() -> (w15469:bool)  [unwired: 1 in]
            n9471 = case shown="True" w15470 {
              tunnel: [TRUE FALSE] -> w15468
              tunnel: w15469 -> [_ w15476]
              tunnel: [FALSE w15473] -> w15465
              frame #0 {
              }
              frame #1 {
                n9472 = call "Elapsed Time184"("Reset"=w15476) -> ("Elapsed Time (s)"=w15475:dbl)  [unwired: 11 in, 7 out]
                n9473 = Greater?(x=w15475, y=5.0) -> (0:w15473:bool)
              }
            }
            n9474 = local write "Trns_gv_bp2_ch1_fail_top"(w15465) -> ()
            n9475 = local write "Trns_gv_bp2_ch1_fail_front"(w15465) -> ()
            n9476 = local write "Ch1_Trns_gv_bp2_fail"(w15465) -> ()
          }
          frame #1 {
            w15478 = TRUE ("Trns_gv_bp2_ch1_fail_front")
            n9477 = local write "Trns_gv_bp2_ch1_fail_top"(w15478) -> ()
            n9478 = local write "Trns_gv_bp2_ch1_fail_front"(w15478) -> ()
            n9479 = local write "Ch1_Trns_gv_bp2_fail"(w15478) -> ()
          }
        }
        n9480 = case shown="False" w15447 {
          frame #0 {
            w15519 = TRUE
            n9481 = local write "Ch1_Ch_vbv_fail"(w15519) -> ()
            n9482 = local write "Ch1_Mp_fail"(w15519) -> ()
            n9483 = local write "Ch1_Tp_bv_fail"(w15519) -> ()
            n9484 = local write "Ch1_Bg_bv_fail"(w15519) -> ()
            n9485 = local write "Ch1_Ch_cc_fail"(w15519) -> ()
            n9486 = local write "ch1_bg_bv_fail_top"(w15519) -> ()
            n9487 = local write "Ch1_Pl_vbv_fail"(w15519) -> ()
            n9488 = local write "Ch1_Pl_atm_fail"(w15519) -> ()
            n9489 = local write "Ch1_Ch_atm_fail"(w15519) -> ()
            n9490 = local write "ch1_cc_fail_top"(w15519) -> ()
            n9491 = local write "ch1_atm_fail_top"(w15519) -> ()
          }
          frame #1 {
            n9492 = local read "Ch1_Mp_do"() -> (w15537:bool)
            n9493 = local read "Ch1_Mp_di"() -> (w15538:bool)
            n9494 = Exclusive Or(1:w15537, 2:w15538) -> (0:w15553:bool)
            n9495 = feedback #323() -> (w15554:bool)  [unwired: 1 in]
            n9496 = case shown="True" w15553 {
              tunnel: [TRUE FALSE] -> w15555
              tunnel: w15554 -> [_ w15596]
              tunnel: [FALSE w15593] -> w15520
              frame #0 {
              }
              frame #1 {
                n9497 = call "Elapsed Time95"("Reset"=w15596) -> ("Elapsed Time (s)"=w15595:dbl)  [unwired: 11 in, 7 out]
                n9498 = Greater?(x=w15595, y=5.0) -> (0:w15593:bool)
              }
            }
            n9499 = local write "Ch1_Mp_fail"(w15520) -> ()